vi "Signal_Schritt für Schritt.vi"(6 "MaxtPeak miltiplication factor":dbl=30.0, 7 "Standard Gap eingeben":dbl=85.0, 8 "Mic.2":dbl[][](array[numeric])=array14x10000[140000 elements], 9 "Mic.1":dbl[][](array[numeric])=array14x10000[140000 elements], 10 "LS auswahlen":i32=13, 11 "Mic. auswählen":bool=TRUE) -> (0 "Array 2":dbl[](array[numeric]), 1 "distanceMatrix":dbl[][](array[numeric]), 2 "Locations":dbl[](array[numeric]), 3 "IR with theshold":dbl[][](graph), 4 "HS":bool, 5 "korriliertes Signal":dbl[](graph))   [LabVIEW 2013]
uses:
  <vilib>/Analysis/3filter.llb/Filter Passband Type.ctl
  <vilib>/Analysis/3filter.llb/Butterworth Filter (DBL).vi
  <vilib>/Analysis/NI_AALBase.lvlib
panel:
  out "Boolesch":bool=TRUE
  in  "correctionValue(samples)":dbl
  in  "Noise Level":dbl=2.0
  in  "RMS miutiplication factor":dbl=2.0
  out "FirstGap":dbl
  # "Envelope with"
  # "Mic. 1"
  # "Mic. 2"
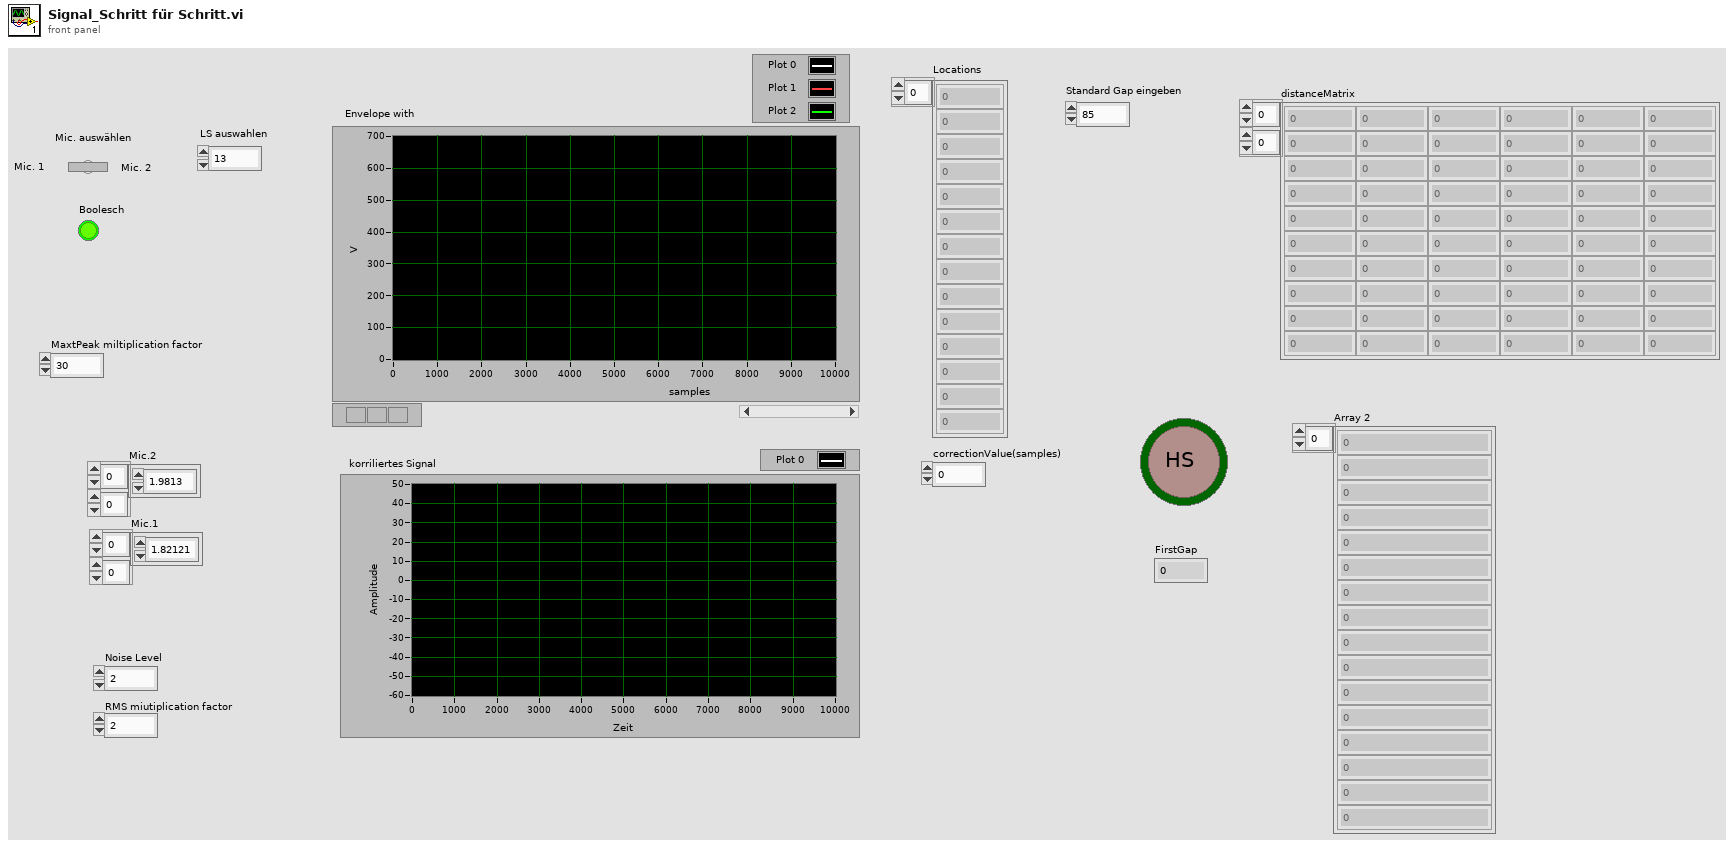
[diagram p1: front panel]
types:
  T1 = typedef "NI_AALBase.lvlib/Filter Passband Type.ctl" = enum32{"Lowpass", "Highpass", "Bandpass", "Bandstop"}
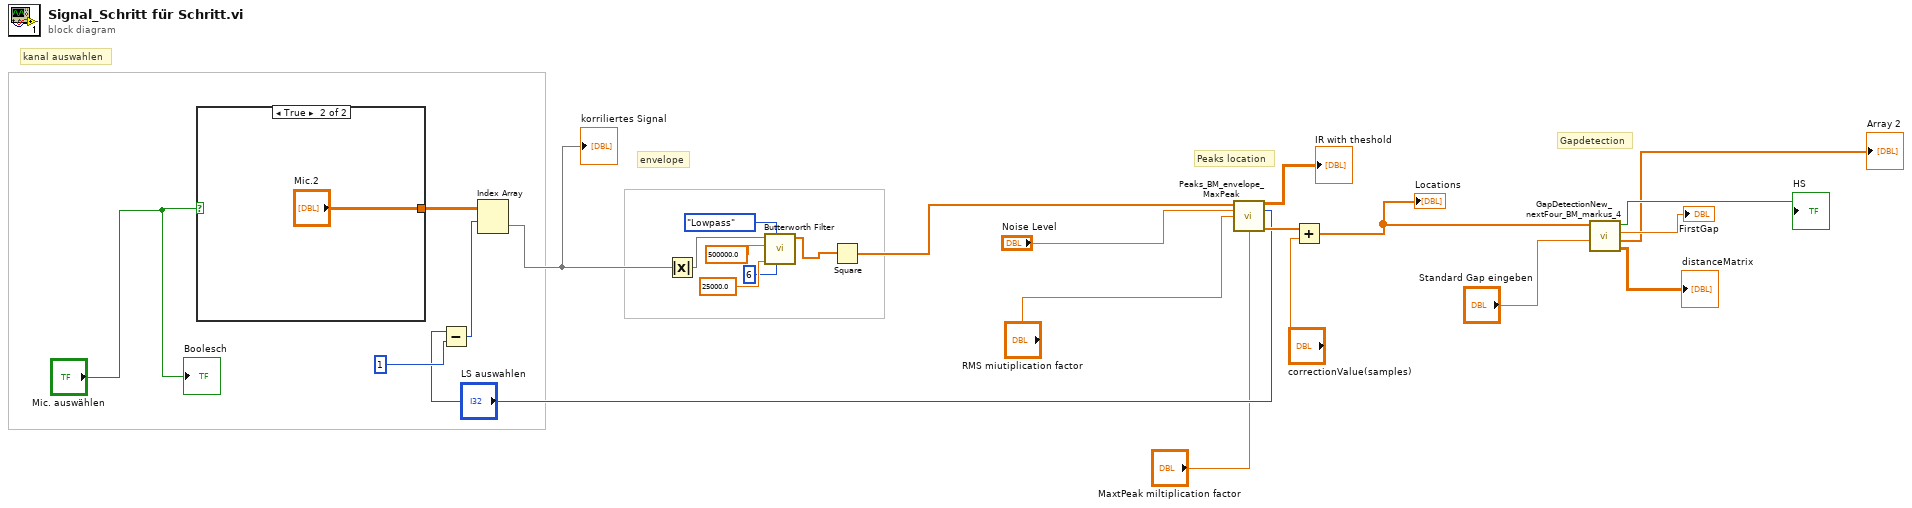
[diagram p0: block diagram]
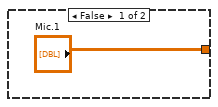
[diagram p2: hidden frame]
diagram:
  # "Gapdetection"
  # "Peaks location"
  # "kanal auswahlen"
  # "envelope"
  n1 = case shown="True" "Mic. auswählen" {
    tunnel: ["Mic.1" "Mic.2"] -> w11
    frame False {
    }
    frame True {
    }
  }
  n2 = Subtract(x="LS auswahlen", y=1) -> (x-y=w6:i32)
  n3 = Index Array(array=w11, index (row)=w6) -> (element=w4:dbl[])  [unwired: 1 in]
  "korriliertes Signal" <- w4
  n4 = Absolute Value(x=w4) -> (abs(x)=w21:dbl[])
  n5 = call-poly <vilib>:"Butterworth Filter.vi"("order"=6, "filter type"=Filter_Passband_Type."Lowpass", "low cutoff freq: fl"=25000.0 ("high cutoff freq: fh"), "sampling freq: fs"=500000.0, "X"=w21) -> ("Filtered X"=w20:dbl[])  [unwired: 3 in, 1 out]
  n6 = Square(x=w20) -> (x^2=w9:dbl[])
  n7 = call "Peaks_BM_envelope_MaxPeak.vi"("imput sequence"=w9, "Noise Level"="Noise Level", "welche LS ?"="LS auswahlen", "RMS miutiplication factor"="RMS miutiplication factor", "MaxPeak miltiplication factor"="MaxtPeak miltiplication factor") -> ("IR with theshold"=→"IR with theshold":dbl[][], "Peak Locations"=w19:dbl[])  [unwired: 8 in, 1 out]
  n8 = Add(x=w19, y="correctionValue(samples)") -> (x+y=w1:dbl[])
  "Locations" <- w1
  n9 = call "GapDetectionNew_nextFour_BM_markus_4.vi"("Gap"="Standard Gap eingeben", "Locations"=w1) -> ("distanceMatrix"=→"distanceMatrix":dbl[][], "Array"=→"Array 2":dbl[], "FirstGap"=→"FirstGap":dbl, "GapPresent"=→"HS":bool)  [unwired: 6 in]
  "Boolesch" <- "Mic. auswählen"
